vi "Joystick and Camera for pattern recognition.vi"(7 "controller in":T1={"A3200.lvclass"=refnum, "Ultimus V2.lvclass"=refnum, "NI-DAQ.lvclass"=refnum, "Motion.lvclass"=refnum, "I-O.lvclass"=refnum, "Dispenser.lvclass"=refnum}, 8 "XYZTheta":dbl[](array[numeric])=[0.026824843572167727, 0.5881986116746664, 0.00020513005945090647, -7.5327256914222e-06], 10 "I-O in":refnum<class "I-O.lvclass">, 11 "Motion in":refnum<class "Motion.lvclass">=refnum) -> (1 "Gantry":dbl[](array[numeric])=[737.9205478380792, 258.97431391859806, 4.360317709278066, -7.264279053542213e-06] format="%#_8g", 2 "I-O out":refnum<class "I-O.lvclass">, 3 "Motion out":refnum<class "Motion.lvclass">, 5 "controller out":T1)   [LabVIEW 2016] (continued)
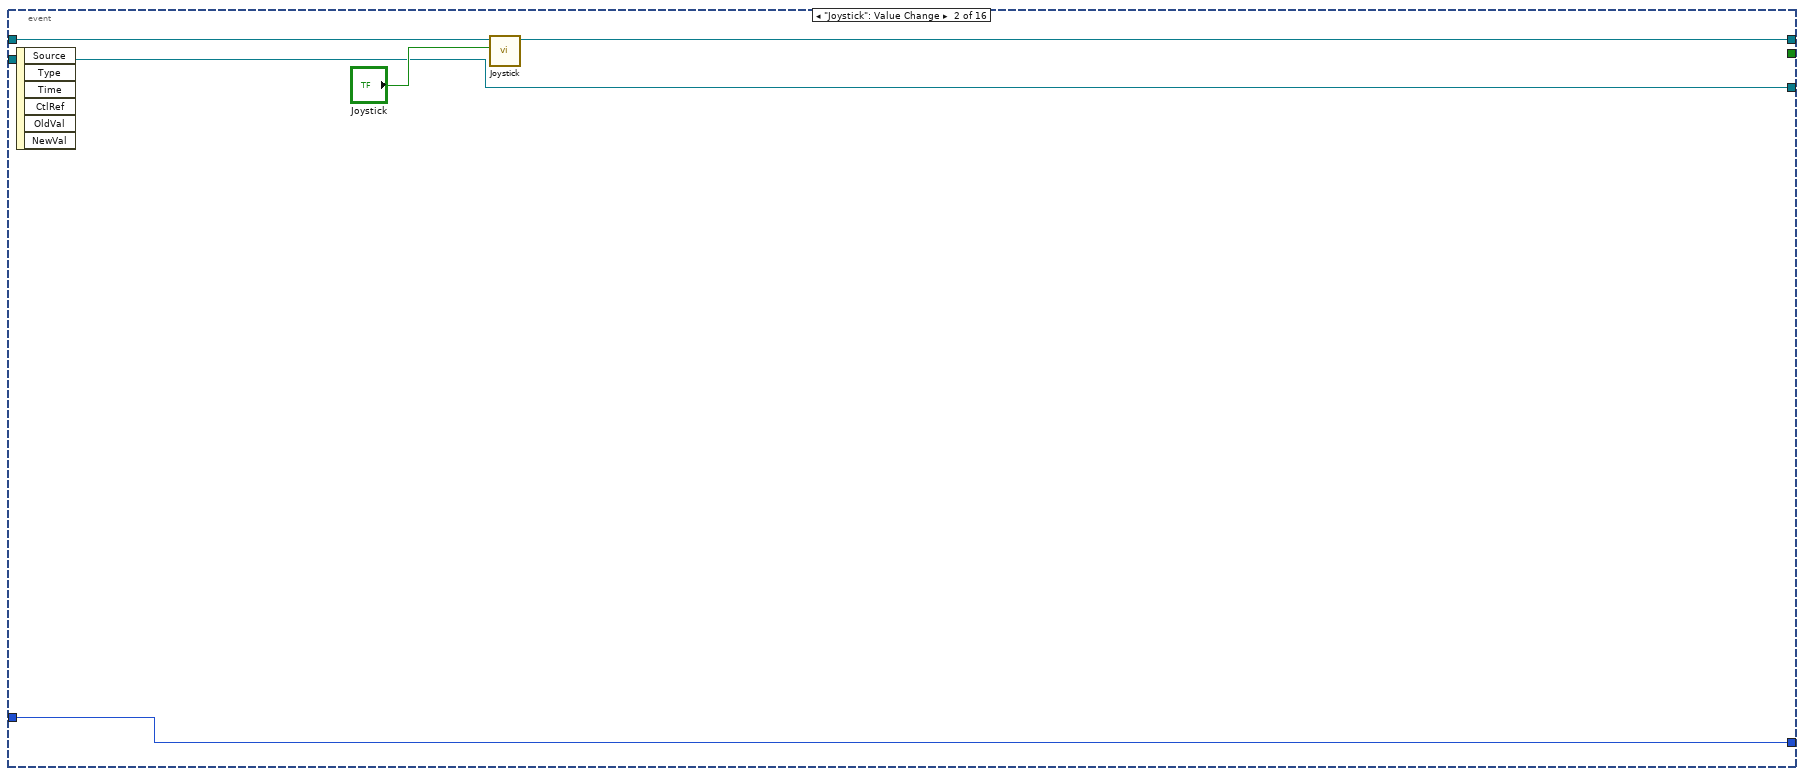
[diagram p3: hidden frame]
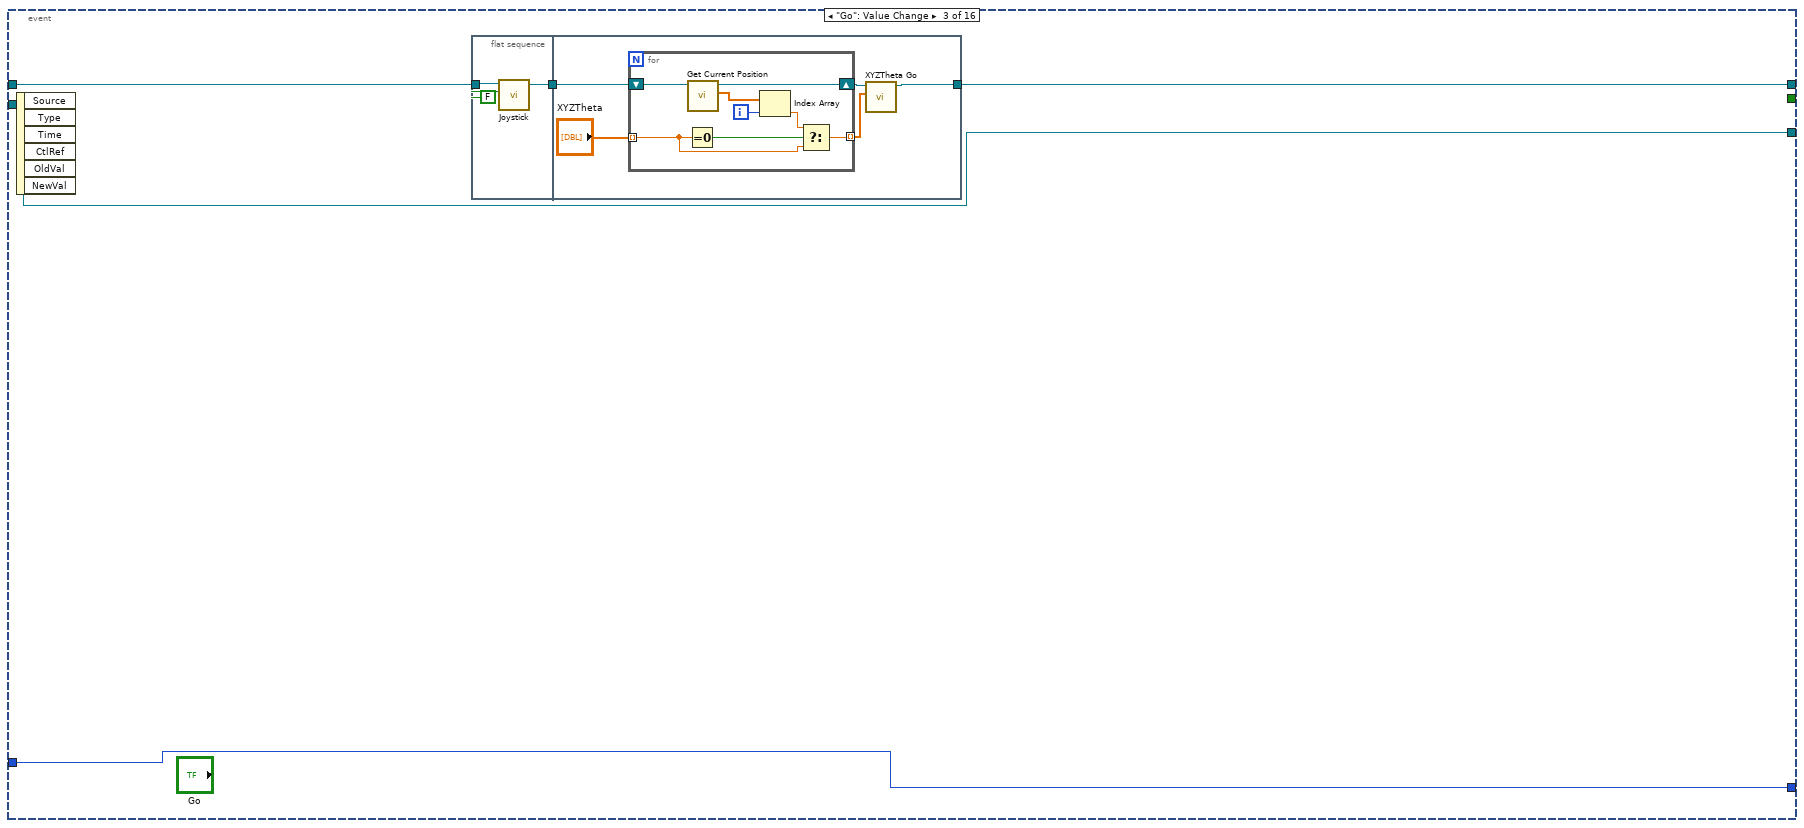
[diagram p4: hidden frame]
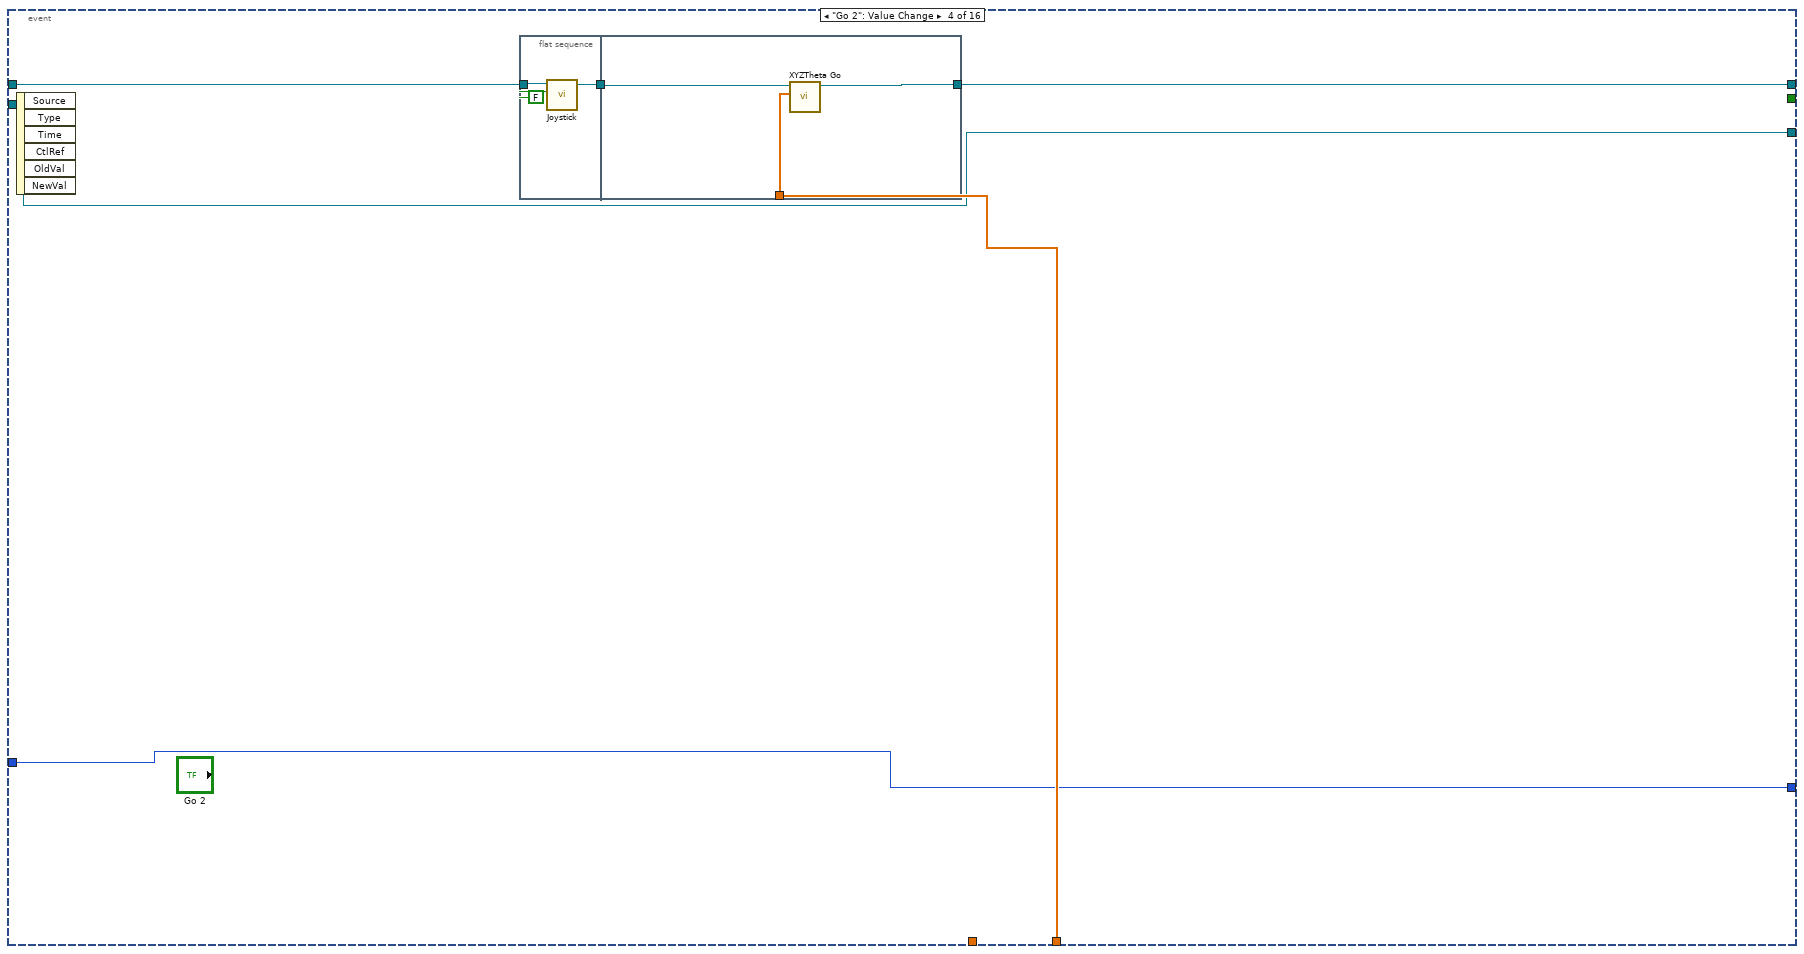
[diagram p5: hidden frame]
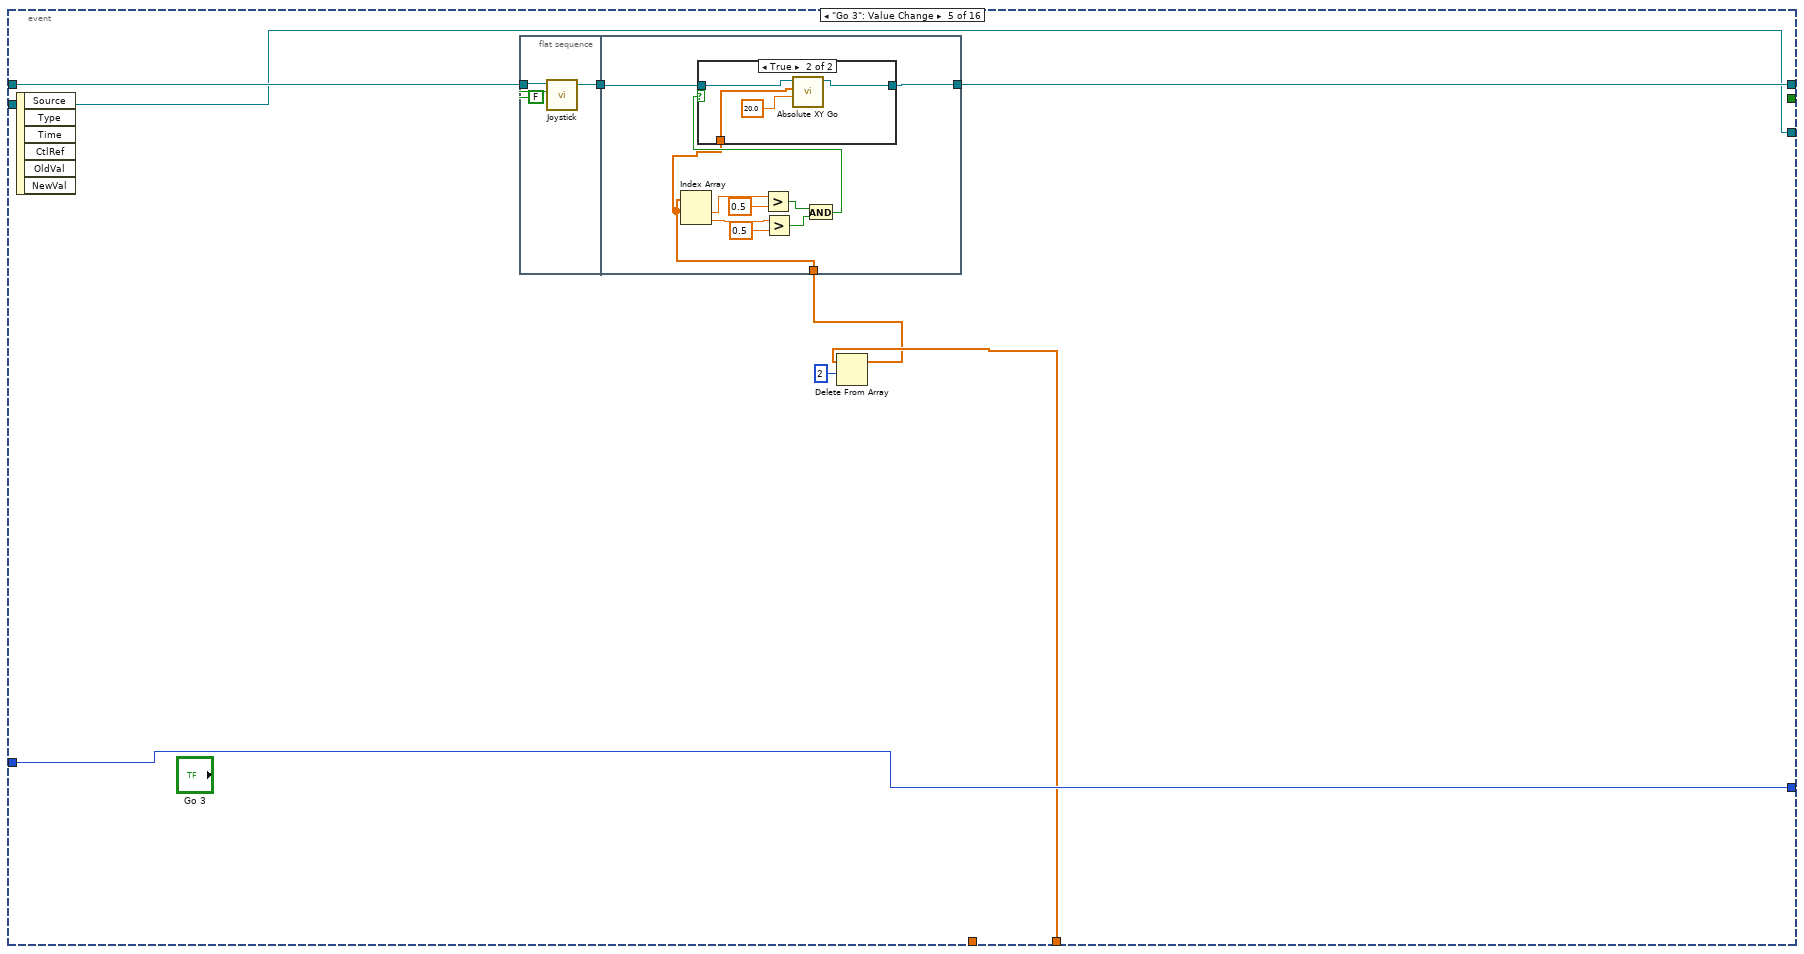
[diagram p6: hidden frame]
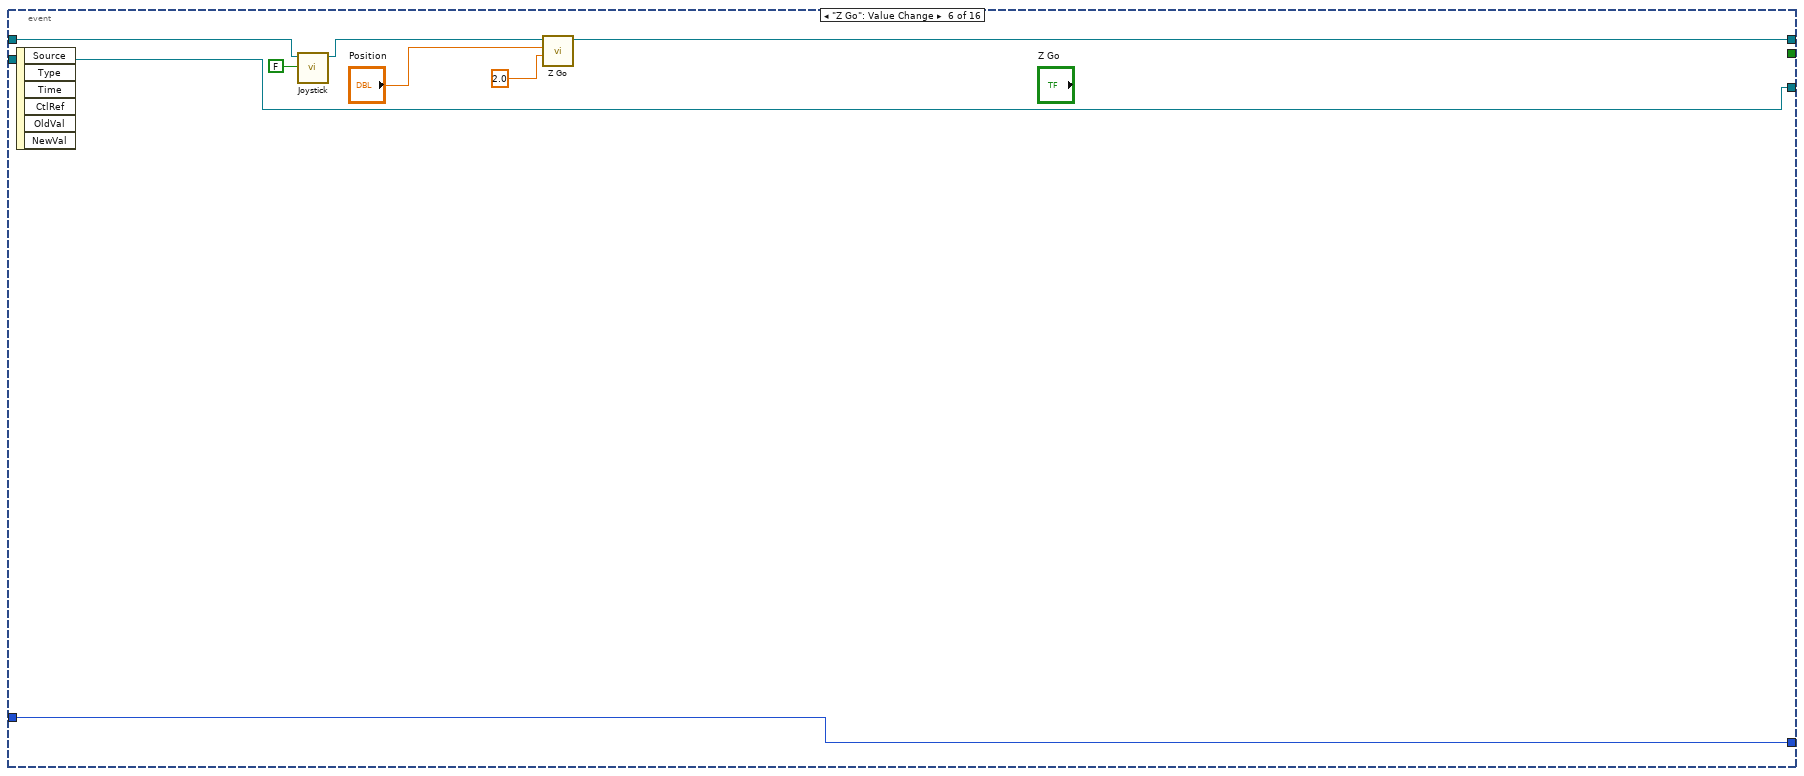
[diagram p8: hidden frame]
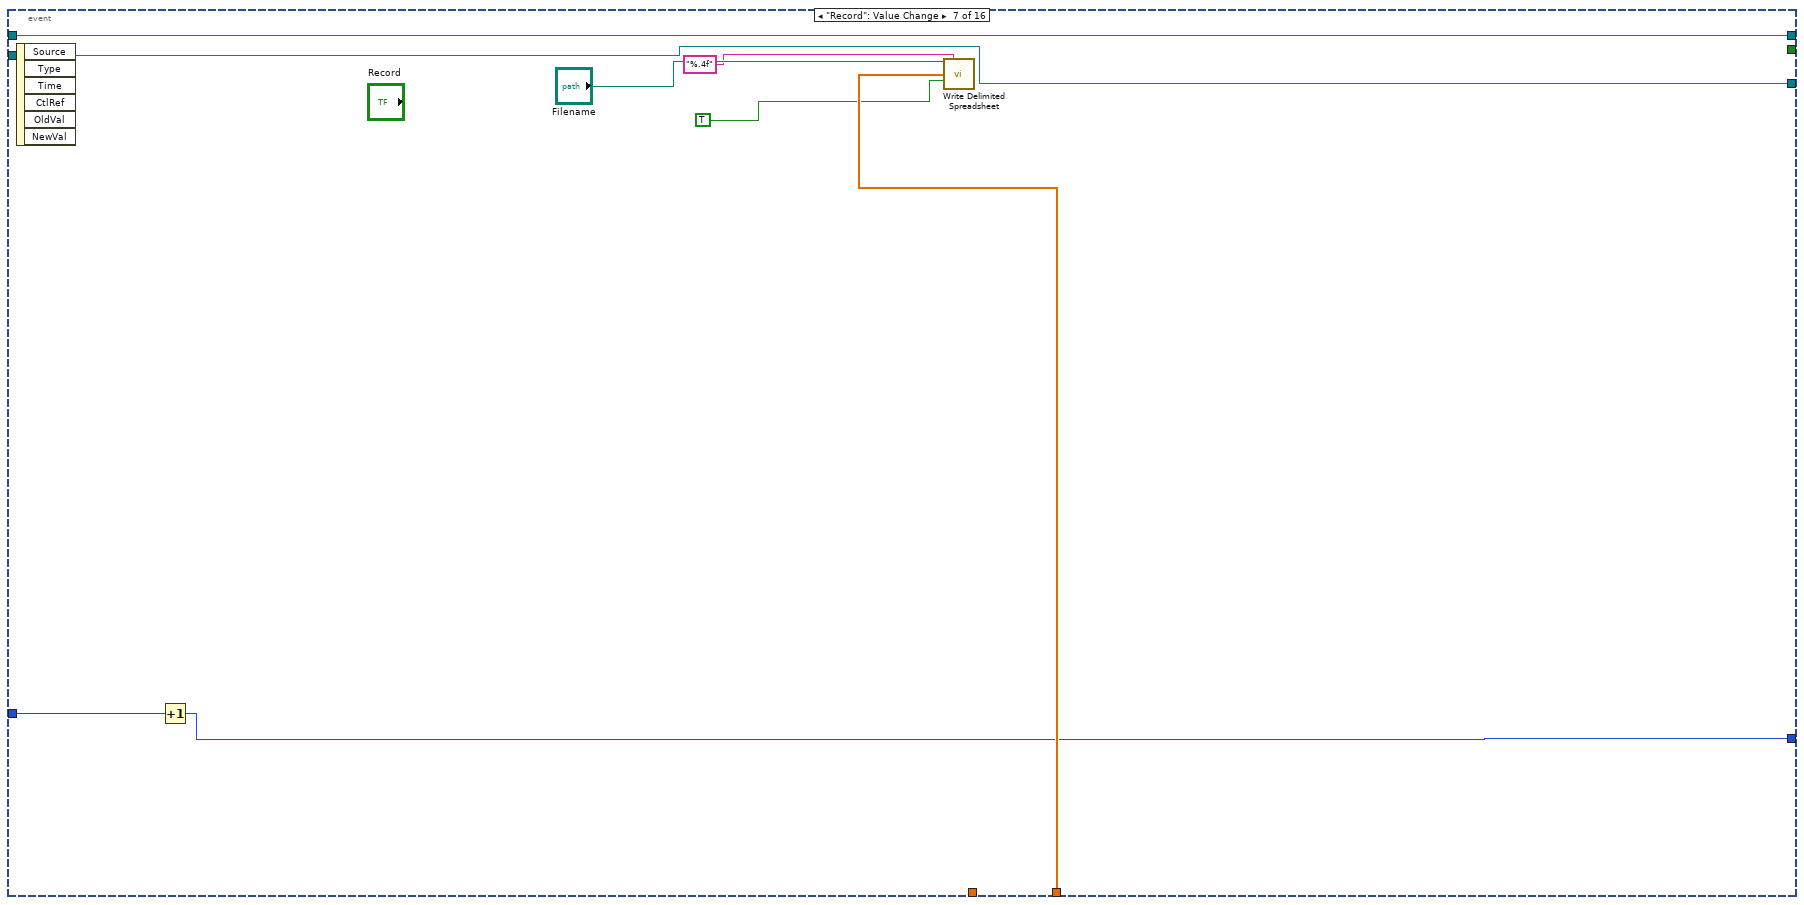
[diagram p9: hidden frame]
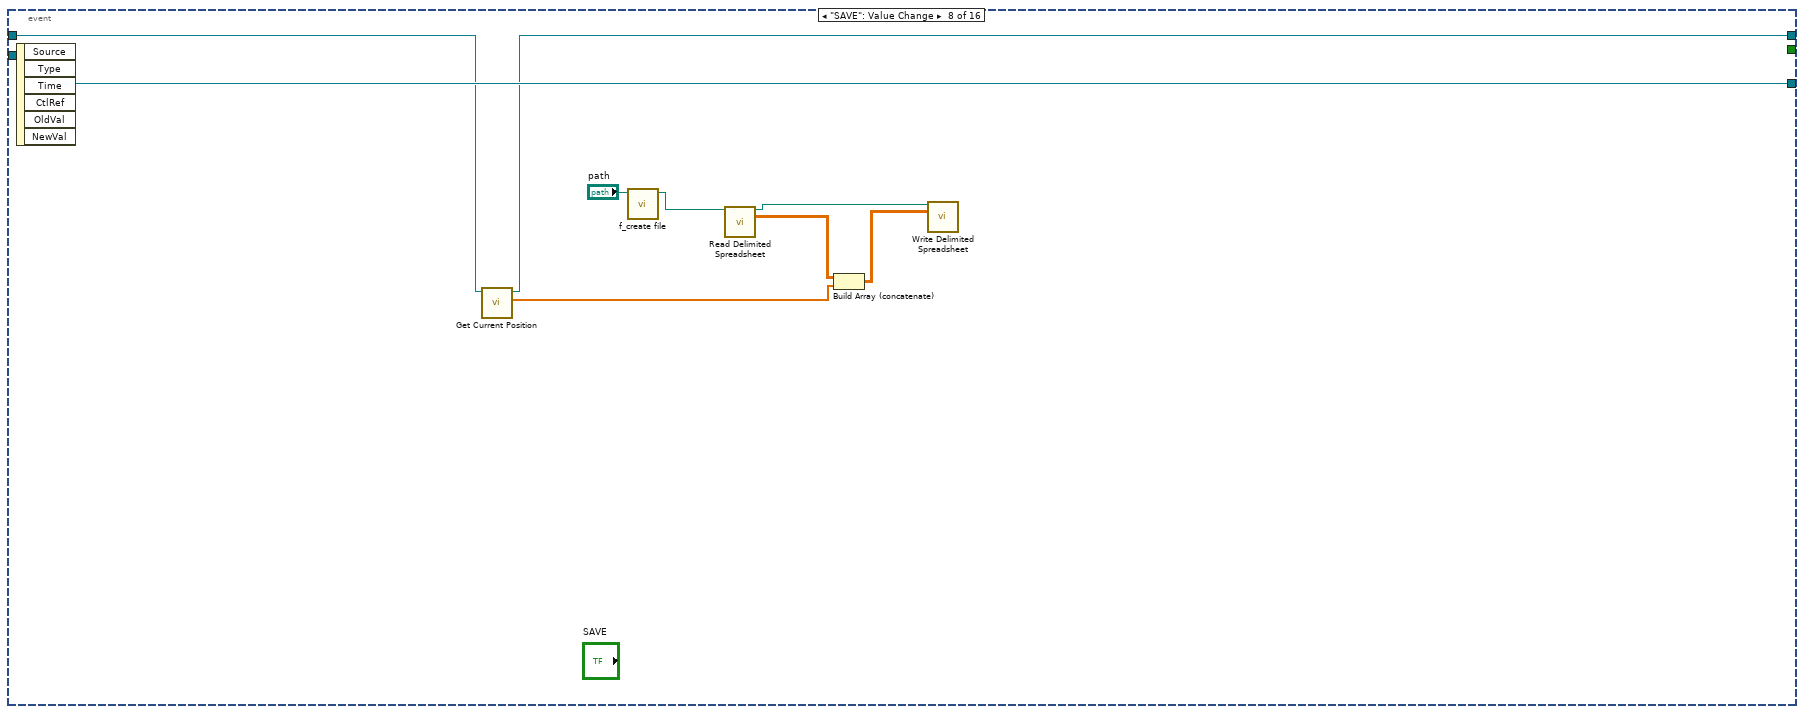
[diagram p10: hidden frame]
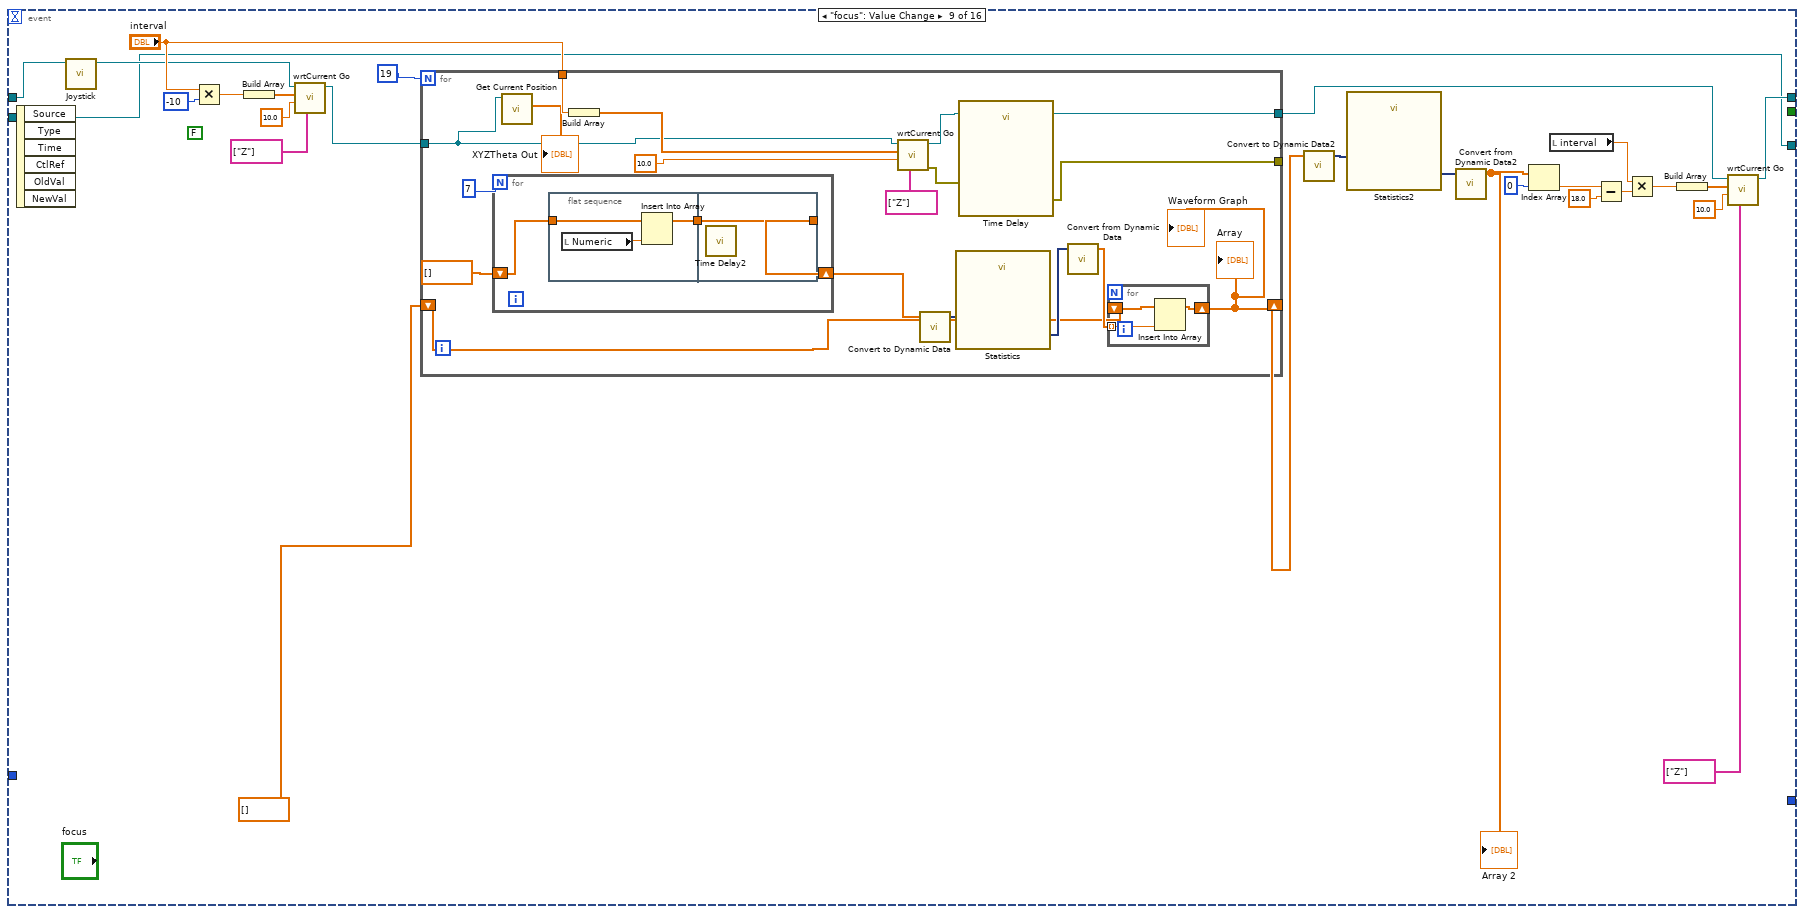
[diagram p11: hidden frame]
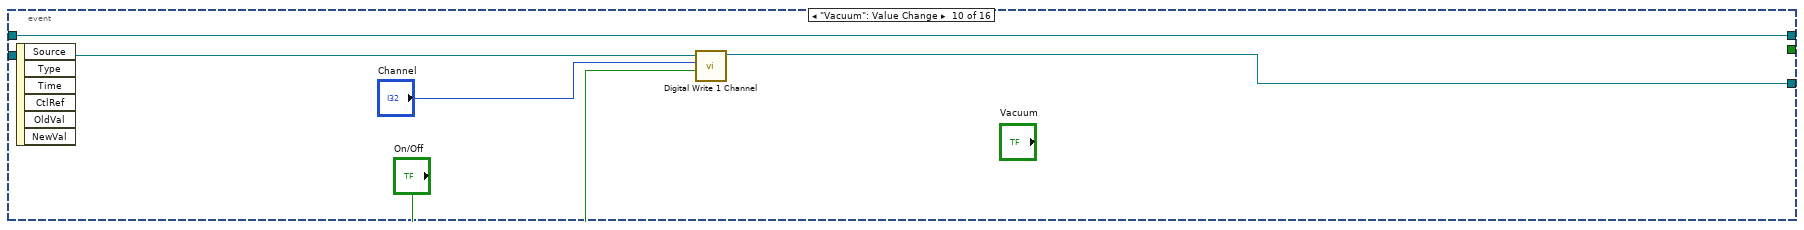
[diagram p12: hidden frame]
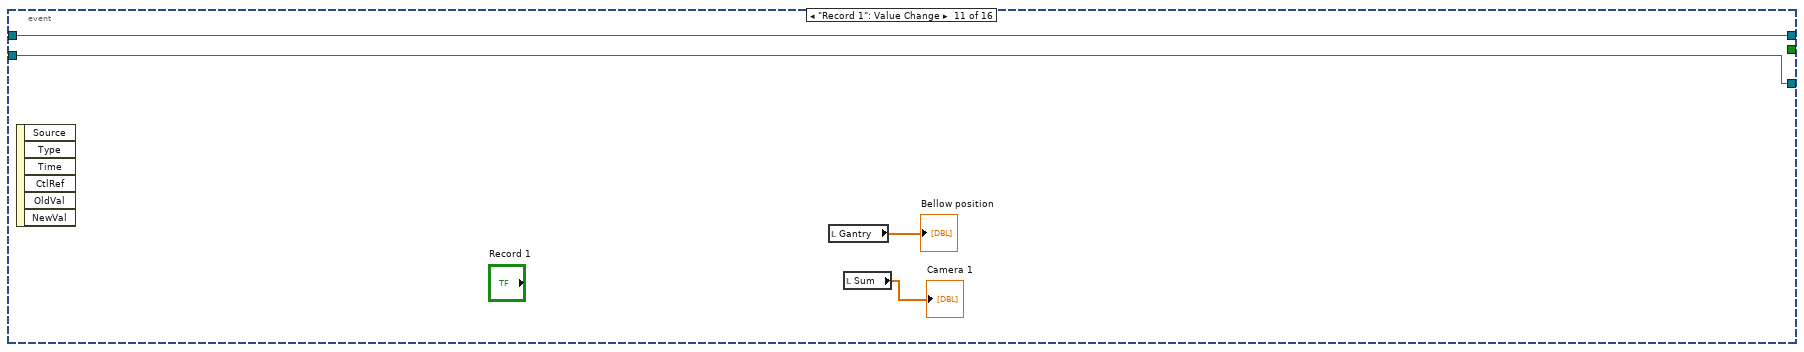
[diagram p13: hidden frame]
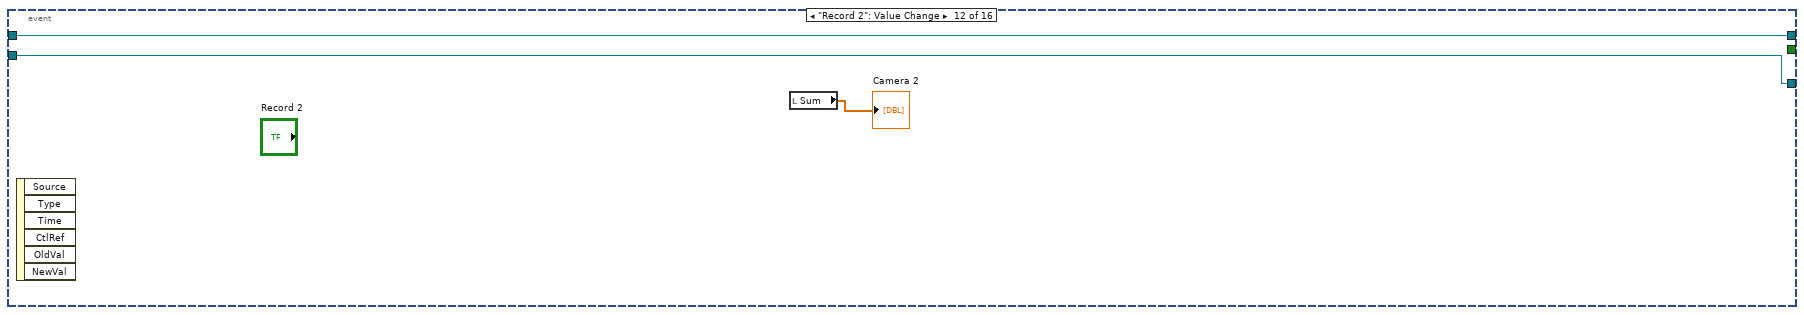
[diagram p14: hidden frame]
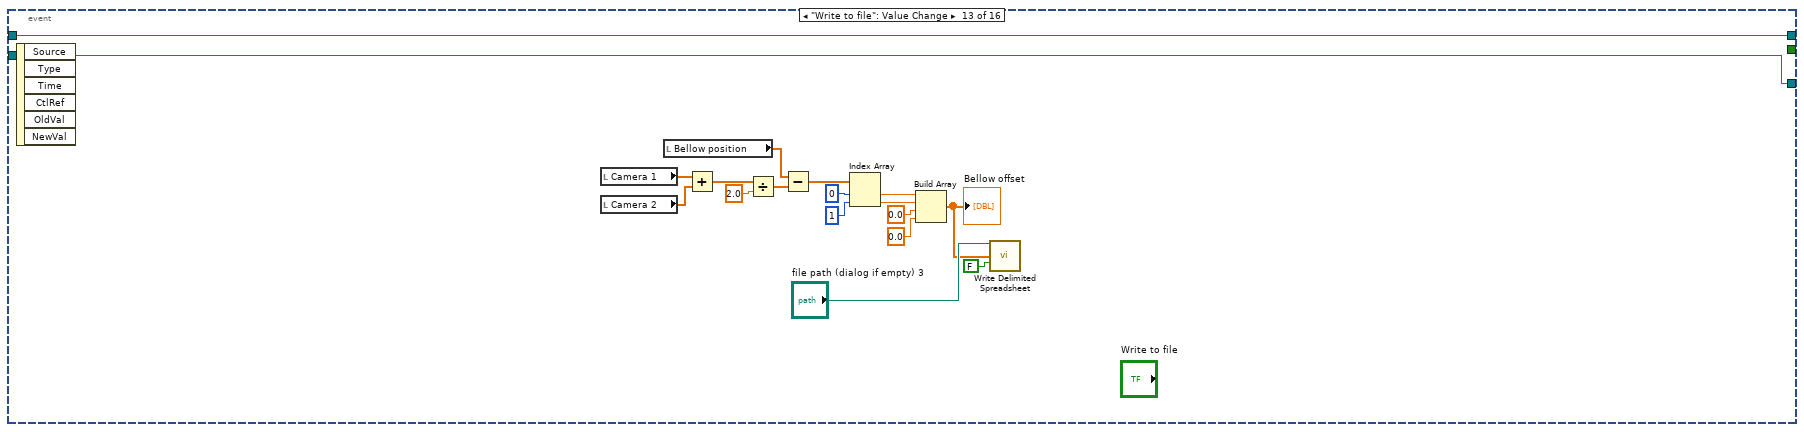
[diagram p15: hidden frame]
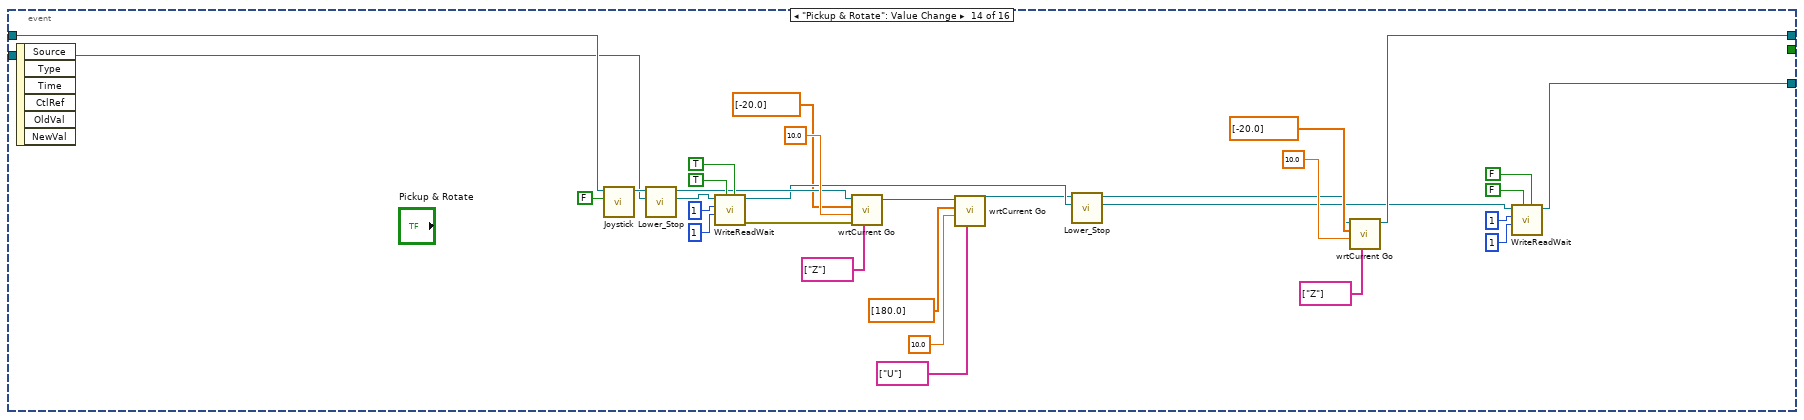
[diagram p16: hidden frame]
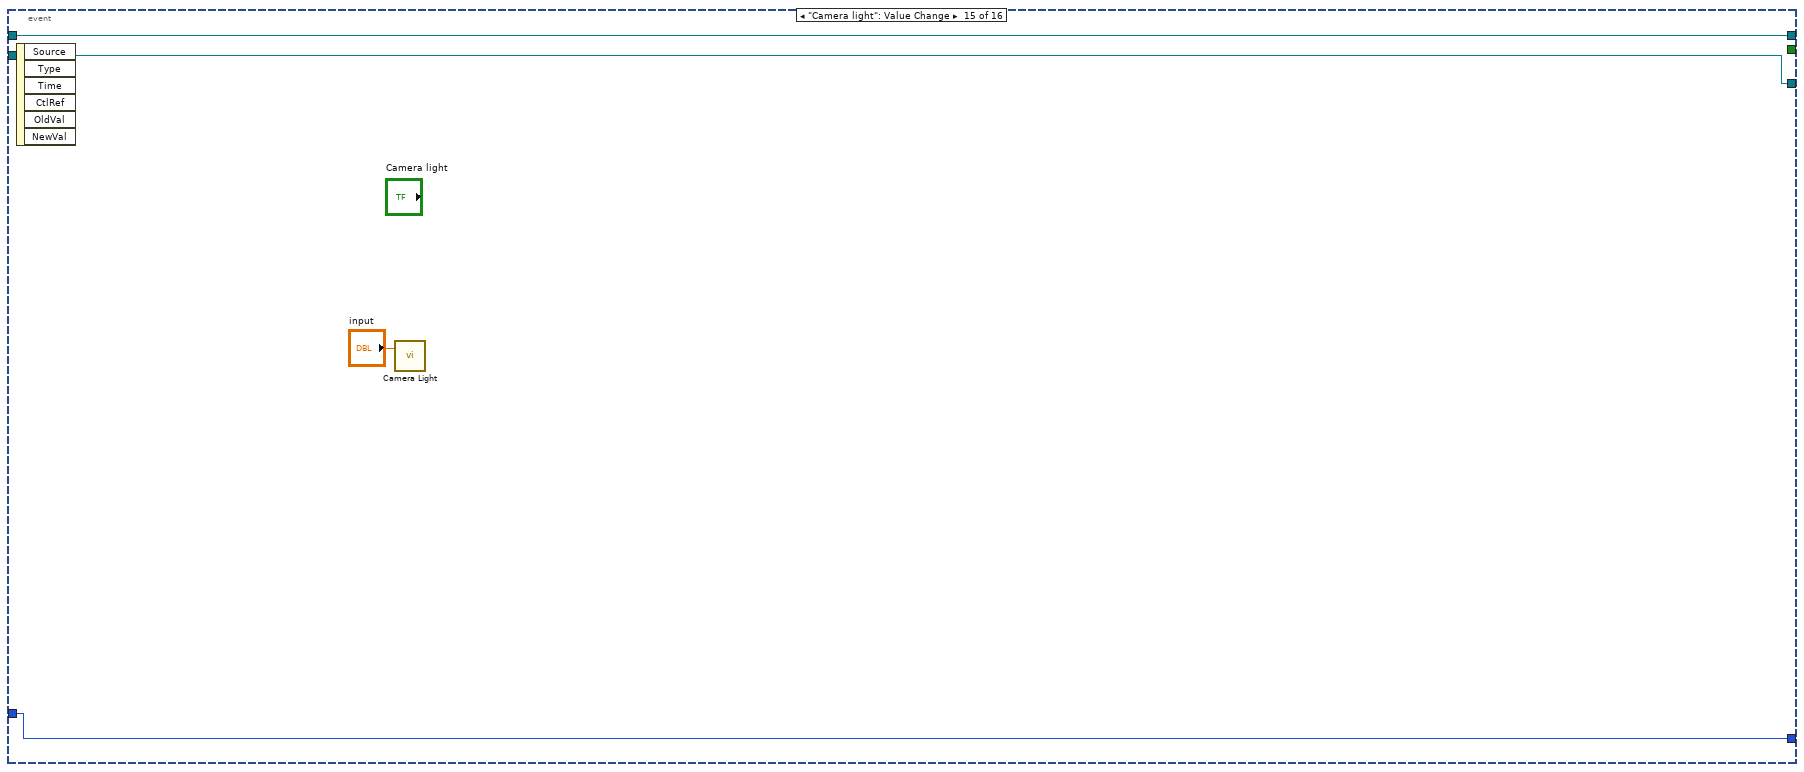
[diagram p17: hidden frame]
